vi "CRYO_MASTER_FULL_IP.vi"() -> ()   [LabVIEW 2017] (continued)
  T22 = cluster{"InstName":string, "Active?":bool, "Status":enum16{"Intialized", "Ready", "Measuring", "Terminated"}, "Labels":string[], "LabelLD":string, "FileFormat":string[], "FileFormatLD":string, "ReadLeakDet?":bool}
  T23 = cluster{"TimeArray":timestamp[], "DataArrayConv":dbl[]}
  T24 = cluster{"TimeArray":timestamp[], "M.A. Array":dbl[]}
  T25 = cluster{"TimeArray":timestamp[], "M.A. Array":dbl[]}[]
  T26 = cluster{"TimeArray":timestamp[], "DataArray":dbl[]}
diagram:
  w9 = TRUE ("create if not found? (T)")
  w15 = errorcluster {"status"=FALSE, "code"=0, "source"=""} ("error in (no error)")
  n1 = while {
    stop <- w44 stop-if-true
    n2 = event shown="[5] \"Plot selecter LSI218(1)     1      2     3     4\", \"Plot selecter LSI218(2)     1      2     3     4\", \"Plot selecter (USB6210)     1      2     3     4\", \"Plot selecter LSI336       1      2     3     4\", \"Plot selecter (USB6218)     1      2     3     4\": Value Change" {
      selector: _ -> [_ _ _ _ _ _ _ _ _ _ _]
      dyn-events: _ -> [_ _ _ _ _ _ _ _ _ _ _]
      timeout: _ -> [_ _ _ _ _ _ _ _ _ _ _]
      tunnel: [_ _ _ _ _ _ _ _ _ _ TRUE] -> w44
      tunnel: [errorcluster {"status"=FALSE, "code"=0, "source"=""} ("error out") w48 _ _ _ _ w178 w195 w212 w229 errorcluster {"status"=FALSE, "code"=0, "source"=""} ("error out")] -> w40
      event Timeout {
        n3 = event-data() -> ()  [unwired: 1 in, 3 out]
      }
      event "log/linear 1": Value Change {
        n4 = event-data() -> ()  [unwired: 1 in, 6 out]
        n5 = flat-sequence {
          tunnel: [w49] -> w48
          frame #0 {
            n6 = control-ref of="Graph 1"() -> (w50:refnum<vi>)
            n7 = Boolean To (0,1)(Boolean="log/linear 1") -> (0, 1=w54:i16)
            n8 = property class="XYGraph (strict)"(reference=w50, error in=errorcluster {"status"=FALSE, "code"=0, "source"=""} ("error in (no error)"), "YScale.Mapping Mode"=w54) -> (error out=w52:errorcluster)  [unwired: 1 out]
            n9 = control-ref of="error out (USB6210)"() -> (w53:refnum<vi>)
            n10 = property class="Clust (strict)"(reference=w53, "Val(Sgnl)"=w52) -> (error out=w49:errorcluster)  [unwired: 1 in, 1 out]
          }
        }
      }
      event "log/linear 2": Value Change {
        n11 = event-data() -> ()  [unwired: 1 in, 6 out]
        n12 = flat-sequence {
          frame #0 {
            n13 = control-ref of="Graph 2"() -> (w58:refnum<vi>)
            n14 = Boolean To (0,1)(Boolean="log/linear 2") -> (0, 1=w60:i16)
            n15 = property class="XYGraph (strict)"(reference=w58, error in=errorcluster {"status"=FALSE, "code"=0, "source"=""} ("error in (no error)"), "YScale.Mapping Mode"=w60) -> (error out=w59:errorcluster)  [unwired: 1 out]
            n16 = control-ref of="error out (USB6210)"() -> (w57:refnum<vi>)
            n17 = property class="Clust (strict)"(reference=w57, "Value"=w59) -> ()  [unwired: 1 in, 2 out]
          }
        }
      }
      event "log/linear 3": Value Change {
        n18 = event-data() -> ()  [unwired: 1 in, 6 out]
        n19 = flat-sequence {
          frame #0 {
            n20 = control-ref of="Graph 3"() -> (w62:refnum<vi>)
            n21 = Boolean To (0,1)(Boolean="log/linear 3") -> (0, 1=w66:i16)
            n22 = property class="XYGraph (strict)"(reference=w62, error in=errorcluster {"status"=FALSE, "code"=0, "source"=""} ("error in (no error)"), "YScale.Mapping Mode"=w66) -> (error out=w65:errorcluster)  [unwired: 1 out]
            n23 = control-ref of="error out (USB6210)"() -> (w64:refnum<vi>)
            n24 = property class="Clust (strict)"(reference=w64, "Value"=w65) -> ()  [unwired: 1 in, 2 out]
          }
        }
      }
      event "log/linear 4": Value Change {
        n25 = event-data() -> ()  [unwired: 1 in, 6 out]
        n26 = flat-sequence {
          frame #0 {
            n27 = control-ref of="Graph 4"() -> (w68:refnum<vi>)
            n28 = Boolean To (0,1)(Boolean="log/linear 4") -> (0, 1=w72:i16)
            n29 = property class="XYGraph (strict)"(reference=w68, error in=errorcluster {"status"=FALSE, "code"=0, "source"=""} ("error in (no error)"), "YScale.Mapping Mode"=w72) -> (error out=w71:errorcluster)  [unwired: 1 out]
            n30 = control-ref of="error out (USB6210)"() -> (w70:refnum<vi>)
            n31 = property class="Clust (strict)"(reference=w70, "Value"=w71) -> ()  [unwired: 1 in, 2 out]
          }
        }
      }
      event "Plot selecter LSI218(1)\n    1      2     3     4", "Plot selecter LSI218(2)\n    1      2     3     4", "Plot selecter (USB6210)\n    1      2     3     4", "Plot selecter LSI336 \n     1      2     3     4", "Plot selecter (USB6218)\n    1      2     3     4": Value Change {
        n32 = event-data() -> ()  [unwired: 1 in, 6 out]
        n33 = local read "All Labels (USB6210)"() -> (w90:string[])
        n34 = local read "All Labels (USB6218)"() -> (w79:string[])
        n35 = local read "Labels LSI218 (1)"() -> (w92:string[])
        n36 = local read "Labels LSI218 (2)"() -> (w93:string[])
        n37 = local read "Labels LSI336"() -> (w85:string[])
        n38 = call "BuildPlotLegends.vi"("Plot selecter \n    1      2     3     4"="Plot selecter (USB6210)\n    1      2     3     4", "AllLabels"=w90) -> ("Series 4"=w102:string[], "Series 3"=w100:string[], "Series 2"=w98:string[], "Series 1"=w96:string[])  [unwired: 6 in]
        n39 = call "BuildPlotLegends_LSI218.vi"("Plot selecter (2)\n    1      2     3     5"="Plot selecter LSI218(2)\n    1      2     3     4", "Plot selecter (1)\n    1      2     3     4"="Plot selecter LSI218(1)\n    1      2     3     4", "Labels (2)"=w93, "Labels (1)"=w92) -> ("Series 4"=w103:string[], "Series 3"=w101:string[], "Series 2"=w99:string[], "Series 1"=w97:string[])  [unwired: 4 in]
        n40 = call "BuildPlotLegends.vi"("Plot selecter \n    1      2     3     4"="Plot selecter LSI336 \n     1      2     3     4", "AllLabels"=w85) -> ("Series 4"=w80:string[], "Series 3"=w81:string[], "Series 2"=w82:string[], "Series 1"=w83:string[])  [unwired: 6 in]
        n41 = call "BuildPlotLegends.vi"("Plot selecter \n    1      2     3     4"="Plot selecter (USB6218)\n    1      2     3     4", "AllLabels"=w79) -> ("Series 4"=w75:string[], "Series 3"=w74:string[], "Series 2"=w76:string[], "Series 1"=w77:string[])  [unwired: 6 in]
        n42 = Build Array (concatenate)(w98, w99, w82, w76) -> (w87:string[])
        "Series 2" <- w87
        n43 = Build Array (concatenate)(w100, w101, w81, w74) -> (w88:string[])
        "Series 3" <- w88
        n44 = Build Array (concatenate)(w102, w103, w80, w75) -> (w89:string[])
        "Series 4" <- w89
        n45 = Build Array (concatenate)(w96, w97, w83, w77) -> (w86:string[])
        "Series 1" <- w86
        n46 = stacked-sequence {
          tunnel: [w113 _ _ _] -> w107
          tunnel: [_ w131 _ _] -> w108
          tunnel: [_ _ w148 _] -> w106
          tunnel: [_ _ _ w165] -> w105
          tunnel: w86 -> [w111 _ _ _]
          tunnel: w87 -> [_ w129 _ _]
          tunnel: w88 -> [_ _ w146 _]
          tunnel: w89 -> [_ _ _ w163]
          frame #0 {
            n47 = Array Size(array=w111) -> (size(s)=w115:i32)
            n48 = control-ref of="Graph 1"() -> (w109:refnum<vi>)
            n49 = property class="XYGraph (strict)"(reference=w109) -> ("LegNumRows"=w110:u32)  [unwired: 1 in, 2 out]
            n50 = for {
              N: w110 -> [_]
              tunnel: w109 -> [w124]
              shift-right: [w122] -> w114
              shift-left: errorcluster {"status"=FALSE, "code"=0, "source"=""} ("error in (no error)") -> [w123]
              i -> [w126]
              n51 = property class="XYGraph (strict)"(reference=w124, error in=w123, "Active Plot"=w126, "Plot.Plot Name"="") -> (error out=w122:errorcluster)  [unwired: 1 out]
            }
            n52 = for {
              N: w115 -> [_]
              tunnel: w109 -> [w120]
              shift-right: [w118] -> w113
              shift-left: w114 -> [w119]
              tunnel: w111 -> [w117] mode=indexing
              i -> [w121]
              n53 = property class="XYGraph (strict)"(reference=w120, error in=w119, "Active Plot"=w121, "Plot.Plot Name"=w117, "Plot.Visible?"=TRUE ("Plot.Visible")) -> (error out=w118:errorcluster)  [unwired: 1 out]
            }
          }
          frame #1 {
            n54 = Array Size(array=w129) -> (size(s)=w133:i32)
            n55 = control-ref of="Graph 2"() -> (w128:refnum<vi>)
            n56 = property class="XYGraph (strict)"(reference=w128) -> ("LegNumRows"=w127:u32)  [unwired: 1 in, 2 out]
            n57 = for {
              N: w127 -> [_]
              shift-right: [w140] -> w132
              shift-left: errorcluster {"status"=FALSE, "code"=0, "source"=""} ("error in (no error)") -> [w141]
              tunnel: w128 -> [w139]
              i -> [w143]
              n58 = property class="XYGraph (strict)"(reference=w139, error in=w141, "Active Plot"=w143, "Plot.Plot Name"="") -> (error out=w140:errorcluster)  [unwired: 1 out]
            }
            n59 = for {
              N: w133 -> [_]
              shift-right: [w136] -> w131
              shift-left: w132 -> [w137]
              tunnel: w129 -> [w135] mode=indexing
              tunnel: w128 -> [w134]
              i -> [w138]
              n60 = property class="XYGraph (strict)"(reference=w134, error in=w137, "Active Plot"=w138, "Plot.Plot Name"=w135) -> (error out=w136:errorcluster)  [unwired: 1 out]
            }
          }
          frame #2 {
            n61 = Array Size(array=w146) -> (size(s)=w150:i32)
            n62 = control-ref of="Graph 3"() -> (w144:refnum<vi>)
            n63 = property class="XYGraph (strict)"(reference=w144) -> ("LegNumRows"=w145:u32)  [unwired: 1 in, 2 out]
            n64 = for {
              N: w145 -> [_]
              tunnel: w144 -> [w158]
              shift-right: [w156] -> w149
              shift-left: errorcluster {"status"=FALSE, "code"=0, "source"=""} ("error in (no error)") -> [w157]
              i -> [w160]
              n65 = property class="XYGraph (strict)"(reference=w158, error in=w157, "Active Plot"=w160, "Plot.Plot Name"="") -> (error out=w156:errorcluster)  [unwired: 1 out]
            }
            n66 = for {
              N: w150 -> [_]
              tunnel: w144 -> [w154]
              shift-right: [w152] -> w148
              shift-left: w149 -> [w153]
              tunnel: w146 -> [w151] mode=indexing
              i -> [w155]
              n67 = property class="XYGraph (strict)"(reference=w154, error in=w153, "Active Plot"=w155, "Plot.Plot Name"=w151) -> (error out=w152:errorcluster)  [unwired: 1 out]
            }
          }
          frame #3 {
            n68 = Array Size(array=w163) -> (size(s)=w167:i32)
            n69 = control-ref of="Graph 4"() -> (w161:refnum<vi>)
            n70 = property class="XYGraph (strict)"(reference=w161) -> ("LegNumRows"=w162:u32)  [unwired: 1 in, 2 out]
            n71 = for {
              N: w162 -> [_]
              tunnel: w161 -> [w175]
              shift-right: [w173] -> w166
              shift-left: errorcluster {"status"=FALSE, "code"=0, "source"=""} ("error in (no error)") -> [w174]
              i -> [w177]
              n72 = property class="XYGraph (strict)"(reference=w175, error in=w174, "Active Plot"=w177, "Plot.Plot Name"="") -> (error out=w173:errorcluster)  [unwired: 1 out]
            }
            n73 = for {
              N: w167 -> [_]
              tunnel: w161 -> [w171]
              shift-right: [w169] -> w165
              shift-left: w166 -> [w170]
              tunnel: w163 -> [w168] mode=indexing
              i -> [w172]
              n74 = property class="XYGraph (strict)"(reference=w171, error in=w170, "Active Plot"=w172, "Plot.Plot Name"=w168) -> (error out=w169:errorcluster)  [unwired: 1 out]
            }
          }
        }
        n75 = Merge Errors(w107, w108, w106, w105) -> (→"Plot errors":errorcluster)
      }
      event "Take Screenshot! 1": Value Change {
        n76 = event-data() -> ()  [unwired: 1 in, 6 out]
        n77 = flat-sequence {
          tunnel: [w179] -> w178
          frame #0 {
            n78 = flat-sequence {
              tunnel: [w180] -> w179
              frame #0 {
                w189 = "_" ("string")
                n79 = local read "RUN Identifier"() -> (w191:string)
                n80 = Get Date/Time In Seconds() -> (seconds since 1Jan1904=w186:timestamp)
                n81 = call "LV_UNIXTIME.vi"("current time"=w186) -> ("date/time string"=w190:string)  [unwired: 9 in, 1 out]
                n82 = control-ref of="Graph 1"() -> (w185:refnum<vi>)
                n83 = Concatenate Strings(w191, w189, w190, w189, "FIle suffix 1", ".png" ("string")) -> (w193:string)
                n84 = local read "Base Path"() -> (w192:path)
                n85 = invoke class="XYGraph (strict)" method="Get Image"(reference=w185, error in=errorcluster {"status"=FALSE, "code"=0, "source"=""} ("error in (no error)")) -> (error out=w181:errorcluster, "image data"=w184:T14)  [unwired: 4 in, 4 out]
                n86 = Build Path(base path=w192, name or relative path=w193) -> (appended path=w183:path)
                n87 = call <vilib>:"Write PNG File.vi"("error in (no error)"=w181, "image data"=w184, "path to PNG file"=w183) -> ("error out"=w180:errorcluster)  [unwired: 7 in, 1 out]
              }
              frame #1 {
                n88 = local write "Take Screenshot! 1"(FALSE ("Take Screenshot! 1")) -> ()
              }
            }
          }
        }
      }
      event "Take Screenshot! 2": Value Change {
        n89 = event-data() -> ()  [unwired: 1 in, 6 out]
        n90 = flat-sequence {
          tunnel: [w196] -> w195
          frame #0 {
            n91 = flat-sequence {
              tunnel: [w202] -> w196
              frame #0 {
                w206 = "_" ("string")
                n92 = local read "RUN Identifier"() -> (w208:string)
                n93 = Get Date/Time In Seconds() -> (seconds since 1Jan1904=w203:timestamp)
                n94 = call "LV_UNIXTIME.vi"("current time"=w203) -> ("date/time string"=w207:string)  [unwired: 9 in, 1 out]
                n95 = control-ref of="Graph 2"() -> (w197:refnum<vi>)
                n96 = Concatenate Strings(w208, w206, w207, w206, "FIle suffix 2", ".png" ("string")) -> (w210:string)
                n97 = local read "Base Path"() -> (w209:path)
                n98 = invoke class="XYGraph (strict)" method="Get Image"(reference=w197, error in=errorcluster {"status"=FALSE, "code"=0, "source"=""} ("error in (no error)")) -> (error out=w201:errorcluster, "image data"=w199:T14)  [unwired: 4 in, 4 out]
                n99 = Build Path(base path=w209, name or relative path=w210) -> (appended path=w198:path)
                n100 = call <vilib>:"Write PNG File.vi"("error in (no error)"=w201, "image data"=w199, "path to PNG file"=w198) -> ("error out"=w202:errorcluster)  [unwired: 7 in, 1 out]
              }
              frame #1 {
                n101 = local write "Take Screenshot! 2"(FALSE ("Take Screenshot! 1")) -> ()
              }
            }
          }
        }
      }
      event "Take Screenshot! 3": Value Change {
        n102 = event-data() -> ()  [unwired: 1 in, 6 out]
        n103 = flat-sequence {
          tunnel: [w213] -> w212
          frame #0 {
            n104 = flat-sequence {
              tunnel: [w215] -> w213
              frame #0 {
                w223 = "_" ("string")
                n105 = local read "RUN Identifier"() -> (w225:string)
                n106 = Get Date/Time In Seconds() -> (seconds since 1Jan1904=w221:timestamp)
                n107 = call "LV_UNIXTIME.vi"("current time"=w221) -> ("date/time string"=w224:string)  [unwired: 9 in, 1 out]
                n108 = control-ref of="Graph 3"() -> (w218:refnum<vi>)
                n109 = Concatenate Strings(w225, w223, w224, w223, "FIle suffix 3", ".png" ("string")) -> (w227:string)
                n110 = local read "Base Path"() -> (w226:path)
                n111 = invoke class="XYGraph (strict)" method="Get Image"(reference=w218, error in=errorcluster {"status"=FALSE, "code"=0, "source"=""} ("error in (no error)")) -> (error out=w216:errorcluster, "image data"=w214:T14)  [unwired: 4 in, 4 out]
                n112 = Build Path(base path=w226, name or relative path=w227) -> (appended path=w219:path)
                n113 = call <vilib>:"Write PNG File.vi"("error in (no error)"=w216, "image data"=w214, "path to PNG file"=w219) -> ("error out"=w215:errorcluster)  [unwired: 7 in, 1 out]
              }
              frame #1 {
                n114 = local write "Take Screenshot! 3"(FALSE ("Take Screenshot! 1")) -> ()
              }
            }
          }
        }
      }
      event "Take Screenshot! 4": Value Change {
        n115 = event-data() -> ()  [unwired: 1 in, 6 out]
        n116 = flat-sequence {
          tunnel: [w230] -> w229
          frame #0 {
            n117 = flat-sequence {
              tunnel: [w233] -> w230
              frame #0 {
                w240 = "_" ("string")
                n118 = local read "RUN Identifier"() -> (w242:string)
                n119 = Get Date/Time In Seconds() -> (seconds since 1Jan1904=w238:timestamp)
                n120 = call "LV_UNIXTIME.vi"("current time"=w238) -> ("date/time string"=w241:string)  [unwired: 9 in, 1 out]
                n121 = control-ref of="Graph 4"() -> (w234:refnum<vi>)
                n122 = Concatenate Strings(w242, w240, w241, w240, "FIle suffix 4", ".png" ("string")) -> (w244:string)
                n123 = local read "Base Path"() -> (w243:path)
                n124 = invoke class="XYGraph (strict)" method="Get Image"(reference=w234, error in=errorcluster {"status"=FALSE, "code"=0, "source"=""} ("error in (no error)")) -> (error out=w231:errorcluster, "image data"=w235:T14)  [unwired: 4 in, 4 out]
                n125 = Build Path(base path=w243, name or relative path=w244) -> (appended path=w236:path)
                n126 = call <vilib>:"Write PNG File.vi"("error in (no error)"=w231, "image data"=w235, "path to PNG file"=w236) -> ("error out"=w233:errorcluster)  [unwired: 7 in, 1 out]
              }
              frame #1 {
                n127 = local write "Take Screenshot! 4"(FALSE ("Take Screenshot! 1")) -> ()
              }
            }
          }
        }
      }
      event "Stop Button": Value Change {
        n128 = event-data() -> ()  [unwired: 1 in, 6 out]
      }
    }
    "error out (graph operations)" <- w40
    n129 = local write "Take Screenshot! 4"(FALSE ("Take Screenshot! 1")) -> ()
    n130 = local write "Take Screenshot! 1"(FALSE ("Take Screenshot! 1")) -> ()
    n131 = local write "Take Screenshot! 2"(FALSE ("Take Screenshot! 1")) -> ()
    n132 = local write "Take Screenshot! 3"(FALSE ("Take Screenshot! 1")) -> ()
    n133 = Wait (ms)(milliseconds to wait=u32 1000) -> ()  [unwired: 1 out]
  }
  n134 = while {
    shift-right: [w256] -> _
    shift-left: refnum<class "6240AData.lvclass"> refnum ("6240AData.lvclass") -> [w254]
    shift-right: [w252] -> _
    shift-left: errorcluster {"status"=FALSE, "code"=0, "source"=""} ("error in (no error)") -> [w253]
    i -> [w248]
    stop <- w255 stop-if-true
    n135 = Wait (ms)(milliseconds to wait=u32 231) -> ()  [unwired: 1 out]
    n136 = Equal?(x=w248, y=0) -> (x = y?=w250:bool)
    n137 = case shown="True" w250 {
      frame False {
      }
      frame True {
        n138 = property on="Initialized?" class="Bool (strict)"("Val(Sgnl)"=FALSE ("Value (Signaling)")) -> ()  [unwired: 2 in, 2 out]
      }
    }
    n139 = event shown="[3] \"Initialize\": Value Change" {
      selector: _ -> [_ _ _ _ _]
      dyn-events: _ -> [_ _ _ _ _]
      timeout: _ -> [_ _ _ _ _]
      tunnel: [w259 w274 _ w323 w344] -> w256
      tunnel: [_ _ _ _ TRUE ("Value (Signaling)")] -> w255
      tunnel: w254 -> [w259 w273 _ w307 w342]
      tunnel: w253 -> [w258 w272 _ w306 w340]
      tunnel: [w258 w271 _ w321 w343] -> w252
      tunnel: w248 -> [_ w270 _ _ _]
      tunnel: w248 -> [_ _ _ w315 _]
      event Timeout {
        n140 = event-data() -> ()  [unwired: 1 in, 3 out]
      }
      event "update values", "SetCurrent 1 (mA)", "SetCurrent 2 (mA)": Value Change {
        w263 = 1000.0 ("y")
        n141 = event-data() -> ()  [unwired: 1 in, 6 out]
        n142 = local read "Initialized?"() -> (w269:bool)
        n143 = Divide(x="SetCurrent 1 (mA)", y=w263) -> (x/y=w264:dbl)
        n144 = Divide(x="SetCurrent 2 (mA)", y=w263) -> (x/y=w265:dbl)
        n145 = Build Array(w264, w265) -> (w262:dbl[])
        n146 = Not Equal?(x=w269, y=FALSE) -> (x != y?=w267:bool)
        n147 = case shown="True" w267 {
          tunnel: [w276 w300] -> w274
          tunnel: "Output\n (ADCMT)" -> [_ w299]
          tunnel: w273 -> [w276 w298]
          tunnel: w272 -> [w275 w297]
          tunnel: [w275 w296] -> w271
          tunnel: w270 -> [_ w292]
          tunnel: w262 -> [_ w278]
          frame False {
          }
          frame True {
            w285 = 1 ("index (col)")
            w286 = 0 ("disabled index (col)")
            n148 = call-dynamic "6240AData_execute.vi"("6240AData in"=w298, "SetCurrent (A)"=w278, "FileFormat"="%3.5f", "Output status"=w299, "ExecutionIndex"=w292, "error in (no error)"=w297) -> ("ActualVoltage (V)"=w277:dbl[], "ActualCurrent (A)"=w291:dbl[], "6240AData out"=w300:refnum<class "6240AData.lvclass">, "appended array"=w281:timestamp[], "SetCurrentArray"=w287:dbl[][], "ActualCurrentArray"=w294:dbl[][], "error out"=w296:errorcluster)  [unwired: 3 in]
            n149 = property on="ActualVoltage (V)" class="Arr (strict)"("Val(Sgnl)"=w277) -> ()  [unwired: 2 in, 2 out]
            n150 = property on="ActualCurrent (A)" class="Arr (strict)"("Val(Sgnl)"=w291) -> ()  [unwired: 2 in, 2 out]
            n151 = Index Array(array=w294, index (col) #1=w286, index (col) #2=w285) -> (element #1=w295:dbl[], element #2=w289:dbl[])  [unwired: 2 in]
            n152 = Index Array(array=w287, index (col) #1=w286, index (col) #2=w285) -> (element #1=w283:dbl[], element #2=w280:dbl[])  [unwired: 2 in]
            n153 = Bundle("appended array"=w281, "ActualCurrentArray"=w295) -> (w290:T15)  [unwired: 1 in]
            n154 = Bundle("appended array"=w281, "ActualCurrentArray"=w289) -> (w284:T15)  [unwired: 1 in]
            n155 = Bundle("appended array"=w281, "SetCurrentArray"=w283) -> (w282:T16)  [unwired: 1 in]
            n156 = Bundle("appended array"=w281, "SetCurrentArray"=w280) -> (w279:T16)  [unwired: 1 in]
            n157 = Build Array(w290, w284, w282, w279) -> (→"Graph 6":T17)
          }
        }
      }
      event "upper limit (mA)", "lower limit (mA)": Value Change {
        n158 = event-data() -> ()  [unwired: 1 in, 6 out]
        n159 = property on="SetCurrent 1 (mA)" class="DigNum (strict)"("Maximum"="upper limit (mA)", "Minimum"="lower limit (mA)") -> ()  [unwired: 2 in, 2 out]
        n160 = property on="SetCurrent 2 (mA)" class="DigNum (strict)"("Maximum"="upper limit (mA)", "Minimum"="lower limit (mA)") -> ()  [unwired: 2 in, 2 out]
      }
      event "Initialize": Value Change {
        w317 = FALSE
        n161 = event-data() -> ()  [unwired: 1 in, 6 out]
        n162 = local read "Initialized?"() -> (w305:bool)
        n163 = case shown="True" w305 {
          tunnel: w307 -> [w333 w337]
          tunnel: w306 -> [w332 w336]
          tunnel: [w333 w335] -> w304
          tunnel: [w332 w334] -> w303
          frame False {
          }
          frame True {
            n164 = call-dynamic "6240AData_terrminate.vi"("error in (no error)"=w336, "6240AData in"=w337) -> ("error out"=w334:errorcluster, "6240AData out"=w335:refnum<class "6240AData.lvclass">)  [unwired: 8 in]
          }
        }
        n165 = property on="Initialized?" class="Bool (strict)"("Val(Sgnl)"=TRUE ("Value (Signaling)")) -> ()  [unwired: 2 in, 2 out]
        n166 = local read "SetCurrent 2 (mA)"() -> (w310:dbl)
        n167 = local read "SetCurrent 1 (mA)"() -> (w313:dbl)
        n168 = local read "RUN Identifier"() -> (w325:string)
        n169 = local read "Base Path"() -> (w326:path)
        n170 = Divide(x=w313, y=1000.0) -> (x/y=w312:dbl)
        n171 = Divide(x=w310, y=1000.0) -> (x/y=w309:dbl)
        n172 = Get Date/Time In Seconds() -> ()  [unwired: 1 out]
        n173 = call-dynamic "6240AData_initialize.vi"("6240AData in"=w304, "RunIdentifier"=w325, "InstName"="InstName", "base path"=w326, "VISA"="VISA", "error in (no error)"=w303, "CtrlLabels"="CtrlLabels", "Voltage limits (V)"="Voltage limits (V)") -> ("6240AData out"=w324:refnum<class "6240AData.lvclass">, "error out"=w322:errorcluster)  [unwired: 6 in]
        n174 = Build Array(w312, w309) -> (w308:dbl[])
        n175 = Build Array(w317, w317) -> (w316:bool[])
        n176 = call-dynamic "6240AData_execute.vi"("6240AData in"=w324, "SetCurrent (A)"=w308, "FileFormat"="%3.5f", "Output status"=w316, "ExecutionIndex"=w315, "error in (no error)"=w322) -> ("ActualVoltage (V)"=w319:dbl[], "ActualCurrent (A)"=w318:dbl[], "6240AData out"=w323:refnum<class "6240AData.lvclass">, "error out"=w321:errorcluster)  [unwired: 3 in, 3 out]
        n177 = property on="ActualVoltage (V)" class="Arr (strict)"("Val(Sgnl)"=w319) -> ()  [unwired: 2 in, 2 out]
        n178 = property on="ActualCurrent (A)" class="Arr (strict)"("Val(Sgnl)"=w318) -> ()  [unwired: 2 in, 2 out]
      }
      event "Stop Button": Value Change {
        n179 = event-data() -> ()  [unwired: 1 in, 6 out]
        n180 = local read "Initialized?"() -> (w338:bool)
        n181 = case shown="False" w338 {
          tunnel: w342 -> [w347 w359]
          tunnel: [w347 w358] -> w341
          tunnel: w340 -> [w346 w357]
          tunnel: [w346 w356] -> w339
          frame False {
          }
          frame True {
            w363 = FALSE
            n182 = local read "SetCurrent 2 (mA)"() -> (w349:dbl)
            n183 = local read "SetCurrent 1 (mA)"() -> (w353:dbl)
            n184 = Divide(x=w353, y=1000.0) -> (x/y=w351:dbl)
            n185 = Divide(x=w349, y=1000.0) -> (x/y=w348:dbl)
            n186 = Build Array(w351, w348) -> (w355:dbl[])
            n187 = Build Array(w363, w363) -> (w354:bool[])
            n188 = property on="Output\n (ADCMT)" class="Arr (strict)"("Val(Sgnl)"=w354) -> ()  [unwired: 2 in, 2 out]
            n189 = call-dynamic "6240AData_execute.vi"("6240AData in"=w359, "SetCurrent (A)"=w355, "FileFormat"="%3.5f", "Output status"=w354, "error in (no error)"=w357) -> ("ActualVoltage (V)"=w360:dbl[], "ActualCurrent (A)"=w361:dbl[], "6240AData out"=w358:refnum<class "6240AData.lvclass">, "error out"=w356:errorcluster)  [unwired: 4 in, 3 out]
            n190 = property on="ActualVoltage (V)" class="Arr (strict)"("Val(Sgnl)"=w360) -> ()  [unwired: 2 in, 2 out]
            n191 = property on="ActualCurrent (A)" class="Arr (strict)"("Val(Sgnl)"=w361) -> ()  [unwired: 2 in, 2 out]
          }
        }
        n192 = call-dynamic "6240AData_terrminate.vi"("error in (no error)"=w339, "6240AData in"=w341) -> ("error out"=w343:errorcluster, "6240AData out"=w344:refnum<class "6240AData.lvclass">)  [unwired: 8 in]
      }
    }
    "error out (ADCMT6420A)" <- w252
  }
  n193 = while {
    shift-right: [w365] -> _
    shift-left: dbl[] [] -> [w371]
    shift-right: [w368] -> _
    shift-left: timestamp[] [] -> [w370]
    i -> [w369]
    stop <- w372 stop-if-true
    n194 = Wait (ms)(milliseconds to wait=u32 225) -> ()  [unwired: 1 out]
    n195 = event shown="[4] \"update current\", \"Set Voltage (V)  (Kikusui)\", \"Set Current (mA)  (Kikusui)\": Value Change" {
      selector: _ -> [_ _ _ _ _ _ _]
      dyn-events: _ -> [_ _ _ _ _ _ _]
      timeout: _ -> [_ _ _ _ _ _ _]
      tunnel: [_ TRUE _ _ _ _ _] -> w372
      tunnel: w369 -> [_ _ _ _ w451 _ _]
      tunnel: [_ _ _ _ w450 w523 _] -> w365
      tunnel: w371 -> [_ _ _ _ w447 w523 _]
      tunnel: [w374 w384 _ _ w449 w522 w528] -> w368
      tunnel: w370 -> [w374 w384 _ _ w448 w522 w528]
      tunnel: w369 -> [_ _ w390 w413 _ _ w529]
      tunnel: [_ _ _ _ w437 _ _] -> w364
      event Timeout {
        n196 = event-data() -> ()  [unwired: 1 in, 3 out]
      }
      event "Stop Button": Value Change {
        w375 = FALSE
        n197 = event-data() -> ()  [unwired: 1 in, 3 out]
        n198 = local read "error out (USB6210/6218 DOUT)"() -> (w383:errorcluster)
        n199 = local read "error out (USB6210/6218 AOUT)"() -> (w380:errorcluster)
        n200 = property on="OUTPUT\n(Kikusui)" class="Bool (strict)"("Value"=w375) -> ()  [unwired: 2 in, 2 out]
        n201 = property on="V2 (N.C.)" class="Bool (strict)"("Val(Sgnl)"=w375) -> ()  [unwired: 2 in, 2 out]
        n202 = local read "DOUT task out"() -> (w379:refnum<k21>)
        n203 = local read "AO task out"() -> (w386:refnum<k21>)
        n204 = Build Array(w375, w375, w375) -> (w382:bool[])
        n205 = Not(x=w375) -> (.not. x?=w376:bool)
        n206 = property on="V1 (N.O.)" class="Bool (strict)"("Val(Sgnl)"=w376) -> ()  [unwired: 2 in, 2 out]
        n207 = call <vilib>:"DAQmx Clear Task.vi"("task in"=w386, "error in"=w380) -> ("error out"=w385:errorcluster)  [unwired: 13 in]
        n208 = local write "error out (USB6210/6218 AOUT)"(w385) -> ()
        n209 = call <vilib>:"DAQmx Write (Digital 1D Bool NChan 1Samp 1Line).vi"("task/channels in"=w379, "data"=w382, "timeout"=10.0, "error in"=w383) -> ("task out"=w378:refnum<k21>, "error out"=w377:errorcluster)  [unwired: 9 in, 1 out]
        n210 = call <vilib>:"DAQmx Clear Task.vi"("task in"=w378, "error in"=w377) -> ("error out"=w387:errorcluster)  [unwired: 13 in]
        n211 = local write "error out (USB6210/6218 DOUT)"(w387) -> ()
      }
      event "V1 (N.O.)": Value Change {
        n212 = event-data() -> ()  [unwired: 1 in, 3 out]
        n213 = local read "Cycle #"() -> (w393:u32)
        n214 = Greater?(x=w393, y=u32 0) -> (0:w391:bool)
        n215 = case shown="True" w391 {
          tunnel: "V1 (N.O.)" -> [_ w406]
          tunnel: w390 -> [_ w401]
          frame False {
          }
          frame True {
            n216 = Not(x=w406) -> (.not. x?=w408:bool)
            n217 = local read "error out (USB6210/6218 DOUT)"() -> (w407:errorcluster)
            n218 = property on="V2 (N.C.)" class="Bool (strict)"() -> ("Value"=w405:bool)  [unwired: 2 in, 2 out]
            n219 = property on="OUTPUT\n(Kikusui)" class="Bool (strict)"() -> ("Value"=w404:bool)  [unwired: 2 in, 2 out]
            n220 = local read "DOUT task out"() -> (w411:refnum<k21>)
            n221 = Build Array(w408, w405, w404) -> (w397:bool[])
            n222 = local read "File Refn USB DO"() -> (w402:refnum<file>)
            n223 = Boolean To (0,1)(Boolean=w397) -> (0, 1=w396:i16[])
            n224 = Initialize Array("%d" ("element"), 3 ("dimension size")) -> (w400:string[])
            n225 = call <vilib>:"DAQmx Write (Digital 1D Bool NChan 1Samp 1Line).vi"("task/channels in"=w411, "data"=w397, "timeout"=10.0, "error in"=w407) -> ("task out"=w409:refnum<k21>, "error out"=w395:errorcluster)  [unwired: 9 in, 1 out]
            n226 = local write "DOUT task out"(w409) -> ()
            n227 = Get Date/Time In Seconds() -> (seconds since 1Jan1904=w403:timestamp)
            n228 = call "FileWrite.vi"("DataArray"=w396, "Time Stamp"=w403, "Error In"=w395, "FileFormat"=w400, "Index"=w401, "refnum in"=w402) -> ("Error Out"=w394:errorcluster)  [unwired: 4 in, 1 out]
            n229 = local write "error out (USB6210/6218 DOUT)"(w394) -> ()
          }
        }
        "V1" <- "V1 (N.O.)"
      }
      event "V2 (N.C.)": Value Change {
        n230 = event-data() -> ()  [unwired: 1 in, 3 out]
        n231 = local read "Cycle #"() -> (w416:u32)
        n232 = Greater?(x=w416, y=u32 0) -> (0:w414:bool)
        n233 = case shown="True" w414 {
          tunnel: "V2 (N.C.)" -> [_ w430]
          tunnel: w413 -> [_ w422]
          frame False {
          }
          frame True {
            n234 = property on="V1 (N.O.)" class="Bool (strict)"() -> ("Value"=w429:bool)  [unwired: 2 in, 2 out]
            n235 = Not(x=w429) -> (.not. x?=w428:bool)
            n236 = local read "error out (USB6210/6218 DOUT)"() -> (w433:errorcluster)
            n237 = property on="OUTPUT\n(Kikusui)" class="Bool (strict)"() -> ("Value"=w427:bool)  [unwired: 2 in, 2 out]
            n238 = local read "DOUT task out"() -> (w434:refnum<k21>)
            n239 = Build Array(w428, w430, w427) -> (w425:bool[])
            n240 = local read "File Refn USB DO"() -> (w426:refnum<file>)
            n241 = Boolean To (0,1)(Boolean=w425) -> (0, 1=w424:i16[])
            n242 = Initialize Array("%d" ("element"), 3 ("dimension size")) -> (w419:string[])
            n243 = call <vilib>:"DAQmx Write (Digital 1D Bool NChan 1Samp 1Line).vi"("task/channels in"=w434, "data"=w425, "timeout"=10.0, "error in"=w433) -> ("task out"=w431:refnum<k21>, "error out"=w418:errorcluster)  [unwired: 9 in, 1 out]
            n244 = local write "DOUT task out"(w431) -> ()
            n245 = Get Date/Time In Seconds() -> (seconds since 1Jan1904=w423:timestamp)
            n246 = call "FileWrite.vi"("DataArray"=w424, "Time Stamp"=w423, "Error In"=w418, "FileFormat"=w419, "Index"=w422, "refnum in"=w426) -> ("Error Out"=w417:errorcluster)  [unwired: 4 in, 1 out]
            n247 = local write "error out (USB6210/6218 DOUT)"(w417) -> ()
          }
        }
        "V2" <- "V2 (N.C.)"
      }
      event "update current", "Set Voltage (V)\n (Kikusui)", "Set Current (mA)\n (Kikusui)": Value Change {
        n248 = event-data() -> ()  [unwired: 1 in, 3 out]
        n249 = case shown="True" "CONTROL KIKUSUI?" {
          tunnel: w451 -> [_ w492]
          tunnel: [w461 w485] -> w450
          tunnel: [w464 w484] -> w449
          tunnel: w448 -> [w466 w487]
          tunnel: w447 -> [w462 w486]
          tunnel: "Set Voltage (V)\n (Kikusui)" -> [_ w477]
          tunnel: "Set Current (mA)\n (Kikusui)" -> [_ w476]
          frame False {
            w463 = 0.0 ("element")
            n250 = Get Date/Time In Seconds() -> (seconds since 1Jan1904=w465:timestamp)
            n251 = local read "AO task out"() -> (w471:refnum<k21>)
            n252 = Build Array (concatenate)(w462, w463) -> (w461:dbl[])
            n253 = Build Array (concatenate)(w466, w465) -> (w464:timestamp[])
            n254 = Build Array(w463, w463) -> (w469:dbl[])
            n255 = call <vilib>:"DAQmx Write (Analog 1D DBL NChan 1Samp).vi"("task/channels in"=w471, "data"=w469, "timeout"=100.0, "error in"=errorcluster {"status"=FALSE, "code"=0, "source"=""}) -> ("task out"=w472:refnum<k21>, "error out"=w467:errorcluster)  [unwired: 9 in, 1 out]
            n256 = local write "AO task out"(w472) -> ()
            n257 = local write "error out (KIKUSI CTRL)"(w467) -> ()
          }
          frame True {
            w474 = 2 ("index")
            (unwired) 2.0 ("y")
            n258 = xnode "Formula"("X1"=w476) -> ("Result"=w481:dbl)  [unwired: 1 in, 1 out]
            n259 = Divide(x=w477, y=650.0) -> (x/y=w499:dbl)
            n260 = Multiply(x=10.0 ("y"), y=w499) -> (x*y=w479:dbl)
            n261 = In Range and Coerce(upper limit=0.4, x=w481, lower limit=0.0 ("y")) -> (coerced(x)=w478:dbl, In Range?=w480:bool)
            n262 = case shown="False" w480 {
              tunnel: w479 -> [w508 w513]
              tunnel: w478 -> [_ w512]
              tunnel: [w506 w511] -> w475
              tunnel: w477 -> [_ w510]
              tunnel: w476 -> [_ w509]
              tunnel: w477 -> [w505 _]
              tunnel: w476 -> [w504 _]
              frame False {
                n263 = Build Array(w505, w504, w508, 0.0 ("element")) -> (w506:dbl[])
              }
              frame True {
                n264 = Build Array(w510, w509, w513, w512) -> (w511:dbl[])
              }
            }
            "USB AOUT" <- w475
            n265 = local read "File Refn USB AO"() -> (w493:refnum<file>)
            n266 = Get Date/Time In Seconds() -> (seconds since 1Jan1904=w488:timestamp)
            n267 = Initialize Array("%.3f", 4 ("dimension size")) -> (w494:string[])
            n268 = local read "AO task out"() -> (w501:refnum<k21>)
            n269 = call "FileWrite.vi"("DataArray"=w475, "Time Stamp"=w488, "Error In"=errorcluster {"status"=FALSE, "code"=0, "source"=""} ("error in"), "FileFormat"=w494, "Index"=w492, "refnum in"=w493) -> ("Error Out"=w490:errorcluster, "Byte Stream File Refnum"=w489:refnum<file>)  [unwired: 4 in]
            n270 = Build Array (concatenate)(w487, w488) -> (w484:timestamp[])
            n271 = local write "File Refn USB AO"(w489) -> ()
            n272 = Array Subset(array=w475, index=w474, length=w474) -> (w473:dbl[])
            n273 = call <vilib>:"DAQmx Write (Analog 1D DBL NChan 1Samp).vi"("task/channels in"=w501, "data"=w473, "timeout"=100.0, "error in"=w490) -> ("task out"=w502:refnum<k21>, "error out"=→"error out (KIKUSI CTRL)":errorcluster)  [unwired: 9 in, 1 out]
            n274 = local write "AO task out"(w502) -> ()
            n275 = Build Array (concatenate)(w486, w476) -> (w485:dbl[])
          }
        }
        n276 = local read "All Labels (USB6218)"() -> (w443:string[])
        n277 = local read "DataArrayConv (USB6218)"() -> (w442:dbl[][])
        n278 = local read "Last Data \n(USB6218)"() -> (w439:dbl[])
        n279 = local read "TimeArray (USB6218)"() -> (w440:timestamp[])
        n280 = Search 1D Array(1D array=w443, element="I_CV") -> (index of element=w444:i32)  [unwired: 1 in]
        n281 = Index Array(array=w442, index (row)=w444) -> (element=w441:dbl[])  [unwired: 1 in]
        n282 = Index Array(array=w439, index=w444) -> (element=w436:dbl)
        n283 = Bundle("TimeArray (USB6218)"=w440, "DataArrayConv (USB6218)"=w441) -> (w437:T18)  [unwired: 1 in]
        n284 = xnode "Formula"("X1"=w436) -> ("Result"=→"Monitor Current (mA)":dbl)  [unwired: 1 in, 1 out]
      }
      event "upper limit (mA)\n (Kikusui)", "upper limit (V)\n (Kikusui)", "lower limit (mA) \n(Kikusui)", "lower limit (V) \n(Kikusui)": Value Change {
        n285 = event-data() -> ()  [unwired: 1 in, 6 out]
        n286 = property on="Set Current (mA)\n (Kikusui)" class="DigNum (strict)"("Maximum"="upper limit (mA)\n (Kikusui)", "Minimum"="lower limit (mA) \n(Kikusui)") -> ()  [unwired: 2 in, 2 out]
        n287 = property on="Set Voltage (V)\n (Kikusui)" class="DigNum (strict)"("Maximum"="upper limit (V)\n (Kikusui)", "Minimum"="lower limit (V) \n(Kikusui)") -> ()  [unwired: 2 in, 2 out]
      }
      event "OUTPUT\n(Kikusui)": Value Change {
        n288 = event-data() -> ()  [unwired: 1 in, 6 out]
        n289 = local read "Cycle #"() -> (w532:u32)
        n290 = Greater?(x=w532, y=u32 0) -> (0:w530:bool)
        n291 = case shown="True" w530 {
          tunnel: w529 -> [_ w536]
          frame False {
          }
          frame True {
            n292 = property on="V1 (N.O.)" class="Bool (strict)"() -> ("Value"=w547:bool)  [unwired: 2 in, 2 out]
            n293 = Not(x=w547) -> (.not. x?=w546:bool)
            n294 = local read "error out (USB6210/6218 DOUT)"() -> (w550:errorcluster)
            n295 = property on="V2 (N.C.)" class="Bool (strict)"() -> ("Value"=w545:bool)  [unwired: 2 in, 2 out]
            n296 = local read "DOUT task out"() -> (w551:refnum<k21>)
            n297 = Build Array(w546, w545, "OUTPUT\n(Kikusui)") -> (w534:bool[])
            n298 = local read "File Refn USB DO"() -> (w537:refnum<file>)
            n299 = Boolean To (0,1)(Boolean=w534) -> (0, 1=w533:i16[])
            n300 = Initialize Array("%d" ("element"), 3 ("dimension size")) -> (w539:string[])
            n301 = call <vilib>:"DAQmx Write (Digital 1D Bool NChan 1Samp 1Line).vi"("task/channels in"=w551, "data"=w534, "timeout"=10.0, "error in"=w550) -> ("task out"=w548:refnum<k21>, "error out"=w541:errorcluster)  [unwired: 9 in, 1 out]
            n302 = local write "DOUT task out"(w548) -> ()
            n303 = Get Date/Time In Seconds() -> (seconds since 1Jan1904=w538:timestamp)
            n304 = call "FileWrite.vi"("DataArray"=w533, "Time Stamp"=w538, "Error In"=w541, "FileFormat"=w539, "Index"=w536, "refnum in"=w537) -> ("Error Out"=w540:errorcluster, "Byte Stream File Refnum"=w535:refnum<file>)  [unwired: 4 in]
            n305 = local write "File Refn USB DO"(w535) -> ()
            n306 = local write "error out (USB6210/6218 DOUT)"(w540) -> ()
          }
        }
      }
    }
    n307 = Bundle(w368, w365) -> (w367:cluster{timestamp[], dbl[]})  [unwired: 1 in]
    n308 = Build Array(w367, w364) -> (→"Graph 7":T9)
  }
  n309 = while {
    stop <- w560 stop-if-true
    n310 = Get Date/Time In Seconds() -> (seconds since 1Jan1904=w559:timestamp)
    n311 = Format Date/Time String(time format string (%c)="%Y%m", seconds (now)=w559) -> (date/time string=w556:string)  [unwired: 1 in]
    n312 = Build Path(base path="Base Path (screenshots)", name or relative path=w556) -> (appended path=w555:path)
    n313 = Create Folder(path (use dialog)=w555, error in=errorcluster {"status"=FALSE, "code"=0, "source"=""}) -> (created path=w552:path, error out=→"error out (monthly folder creation)":errorcluster)  [unwired: 1 in, 1 out]
    n314 = event shown="[1] \"Frontpanel screenshots\": Value Change" {
      selector: _ -> [_ _ _]
      dyn-events: _ -> [_ _ _]
      timeout: _ -> [_ _ _]
      tunnel: [FALSE _ TRUE] -> w560
      tunnel: w552 -> [_ w568 _]
      tunnel: w559 -> [_ w567 _]
      event Timeout {
        n315 = event-data() -> ()  [unwired: 1 in, 3 out]
      }
      event "Frontpanel screenshots": Value Change {
        n316 = event-data() -> ()  [unwired: 1 in, 3 out]
        n317 = property class="TabCtl (strict)"() -> ("Value"=w565:T2)  [unwired: 2 in, 2 out]
        n318 = stacked-sequence {
          tunnel: w568 -> [w574 w596 w618 w640 w662 w684 w706 w728 _]
          tunnel: w567 -> [w573 w595 w617 w639 w661 w683 w705 w727 _]
          tunnel: [w571 _ _ _ _ _ _ _ _] -> w566
          tunnel: w565 -> [w570 _ _ _ _ _ _ _ _]
          tunnel: [w570 _ _ _ _ _ _ _ _] -> w564
          tunnel: "cryostatus_" ("string") -> [w569 w592 w614 w636 w658 w680 w702 w724 _]
          frame #0 {
            n319 = flat-sequence {
              tunnel: w573 -> [w576]
              tunnel: [w576] -> w572
              tunnel: w574 -> [w591]
              tunnel: w572 -> [w579]
              tunnel: [w578] -> w571
              tunnel: w569 -> [w577]
              frame #0 {
                n320 = property class="TabCtl (strict)"("Val(Sgnl)"=T2."NI USB CONFIG" ("Value (Signaling)")) -> ()  [unwired: 2 in, 2 out]
              }
              frame #1 {
                w589 = "_" ("string")
                n321 = local read "Cycle #"() -> (w587:u32)
                n322 = call "LV_UNIXTIME.vi"("current time"=w579) -> ("date/time string"=w590:string)  [unwired: 9 in, 1 out]
                n323 = Format Value(format string="%06d", value (0)=w587) -> (output string=w586:string)  [unwired: 1 in]
                n324 = Concatenate Strings(w577, w590, w589, w586, w589, "page1.png" ("string")) -> (w584:string)